vi "Dresden R2R Sputter 03.02.2018 IY24.vi"() -> ()   [LabVIEW 2009] (continued)
                                n31208 = case shown="False" w35965 {
                                tunnel: [FALSE TRUE] -> w35963
                                frame #0 {
                                n31209 = Wait Until Next ms Multiple(millisecond multiple=u32 200) -> ()  [unwired: 1 out]
                                }
                                frame #1 {
                                }
                                }
                                n31210 = Or(x=w35963, y=w35964) -> (x .or. y?=w35962:bool)
                                }
                                }
                                frame #1 {
                                }
                                }
                                }
                                frame #4 {
                                n31211 = local read "Semi"() -> (w35975:bool)
                                n31212 = case shown="False" w35975 {
                                frame #0 {
                                n31213 = local read "Set_pressure_value 2"() -> (w35976:dbl)
                                n31214 = Add(x=1.0, y=w35976) -> (x+y=w35979:dbl)
                                n31215 = Subtract(x=w35976, y=1.0) -> (x-y=w35980:dbl)
                                n31216 = local read "Pressure 2"() -> (w35977:i32)
                                n31217 = In Range and Coerce(upper limit=w35979, x=w35977, lower limit=w35980) -> (In Range?=w35978:bool)  [unwired: 1 out]
                                n31218 = case shown="False" w35978 {
                                frame #0 {
                                n31219 = local read "R Set Pressure mtorr"() -> (w35983:dbl)
                                n31220 = local write "Set_pressure_value 2"(w35983) -> ()
                                }
                                frame #1 {
                                }
                                }
                                }
                                frame #1 {
                                }
                                }
                                }
                                frame #5 {
                                n31221 = local read "Semi"() -> (w35984:bool)
                                n31222 = case shown="False" w35984 {
                                frame #0 {
                                n31223 = local read "Set_pressure_value 2"() -> (w35985:dbl)
                                n31224 = Add(x=1.0, y=w35985) -> (x+y=w35988:dbl)
                                n31225 = Subtract(x=w35985, y=1.0) -> (x-y=w35989:dbl)
                                n31226 = local read "Pressure 2"() -> (w35986:i32)
                                n31227 = In Range and Coerce(upper limit=w35988, x=w35986, lower limit=w35989) -> (In Range?=w35987:bool)  [unwired: 1 out]
                                n31228 = case shown="False" w35987 {
                                frame #0 {
                                n31229 = local write "Pc_bv2_auto_set_pressure"(TRUE ("Pc_bv1_auto_set_pressure")) -> ()
                                }
                                frame #1 {
                                }
                                }
                                }
                                frame #1 {
                                }
                                }
                                }
                                frame #6 {
                                n31230 = local read "Semi"() -> (w35993:bool)
                                n31231 = case shown="False" w35993 {
                                frame #0 {
                                n31232 = while {
                                i -> [w36004]
                                stop <- w35995 stop-if-true
                                n31233 = local read "Set_pressure_value 2"() -> (w35999:dbl)
                                n31234 = Greater?(x=w36004, y=300) -> (0:w35997:bool)
                                n31235 = Add(x=1.0, y=w35999) -> (x+y=w36000:dbl)
                                n31236 = Subtract(x=w35999, y=1.0) -> (x-y=w36001:dbl)
                                n31237 = local read "Pressure 2"() -> (w35994:i32)
                                n31238 = In Range and Coerce(upper limit=w36000, x=w35994, lower limit=w36001) -> (In Range?=w35998:bool)  [unwired: 1 out]
                                n31239 = case shown="False" w35998 {
                                tunnel: [FALSE TRUE] -> w35996
                                frame #0 {
                                n31240 = Wait Until Next ms Multiple(millisecond multiple=u32 200) -> ()  [unwired: 1 out]
                                }
                                frame #1 {
                                }
                                }
                                n31241 = Or(x=w35996, y=w35997) -> (x .or. y?=w35995:bool)
                                }
                                }
                                frame #1 {
                                }
                                }
                                }
                                frame #7 {
                                n31242 = local read "Semi"() -> (w36009:bool)
                                n31243 = case shown="False" w36009 {
                                frame #0 {
                                n31244 = local read "Set_pressure_value 2"() -> (w36012:dbl)
                                n31245 = Add(x=1.0, y=w36012) -> (x+y=w36013:dbl)
                                n31246 = Subtract(x=w36012, y=1.0) -> (x-y=w36014:dbl)
                                n31247 = local read "Pressure 2"() -> (w36010:i32)
                                n31248 = In Range and Coerce(upper limit=w36013, x=w36010, lower limit=w36014) -> (In Range?=w36011:bool)  [unwired: 1 out]
                                n31249 = case shown="False" w36011 {
                                frame #0 {
                                n31250 = local write "Semi"(TRUE ("Semi")) -> ()
                                n31251 = local write "Error Message"("Coating Pressure could not be adjusted !" ("Error Message")) -> ()
                                }
                                frame #1 {
                                }
                                }
                                }
                                frame #1 {
                                }
                                }
                                }
                                }
                                }
                                frame #1 {
                                }
                                }
                                }
                                frame #1 {
                                n31252 = local read "Semi"() -> (w36019:bool)
                                n31253 = case shown="False" w36019 {
                                frame #0 {
                                n31254 = local write "SDC1 9"(TRUE ("SDC1 9")) -> ()
                                n31255 = Wait (ms)(milliseconds to wait=u32 1000) -> ()  [unwired: 1 out]
                                }
                                frame #1 {
                                }
                                }
                                }
                                }
                                }
                                }
                                }
                                frame #1 {
                                }
                                }
                                }
                                frame #13 {
                                n31256 = local read "Semi"() -> (w36022:bool)
                                n31257 = case shown="False" w36022 {
                                frame #0 {
                                n31258 = local write "Start_roll"(TRUE ("Start_roll")) -> ()
                                n31259 = Wait (ms)(milliseconds to wait=u32 300) -> ()  [unwired: 1 out]
                                }
                                frame #1 {
                                }
                                }
                                }
                                frame #14 {
                                n31260 = local read "Semi"() -> (w36025:bool)
                                n31261 = case shown="False" w36025 {
                                frame #0 {
                                n31262 = local read "R Cmb Ch2 Step1 Coating Power Active"() -> (w36036:bool)
                                n31263 = local read "R Cmb Ch2 Step2 Coating Power Active"() -> (w36035:bool)
                                n31264 = local read "R Cmb Ch2 Step3 Coating Power Active"() -> (w36034:bool)
                                n31265 = local read "R Cmb Ch2 Step4 Coating Power Active"() -> (w36033:bool)
                                n31266 = local read "R Cmb Ch2 Step5 Coating Power Active"() -> (w36032:bool)
                                n31267 = Boolean To (0,1)(Boolean=w36036) -> (0, 1=w36031:i16)
                                n31268 = Boolean To (0,1)(Boolean=w36035) -> (0, 1=w36030:i16)
                                n31269 = Boolean To (0,1)(Boolean=w36034) -> (0, 1=w36029:i16)
                                n31270 = Boolean To (0,1)(Boolean=w36033) -> (0, 1=w36028:i16)
                                n31271 = Boolean To (0,1)(Boolean=w36032) -> (0, 1=w36027:i16)
                                n31272 = Compound Arithmetic op=ADD(w36031, w36030, w36029, w36028, w36027) -> (w36026:i16)
                                n31273 = case shown="5" w36026 {
                                frame #0 {
                                }
                                frame #1 {
                                n31274 = stacked-sequence {
                                frame #0 {
                                n31275 = local read "R Cmb Ch2 Step1 Coating Power Active"() -> (w36037:bool)
                                n31276 = case shown="True" w36037 {
                                frame #0 {
                                }
                                frame #1 {
                                n31277 = while {
                                stop <- w36039 stop-if-true
                                n31278 = local read "R Cmb Interval length"() -> (w36043:dbl)
                                n31279 = local read "Actual Length"() -> (w36042:dbl)
                                n31280 = Greater Or Equal?(x=w36042, y=w36043) -> (x >= y?=w36041:bool)
                                n31281 = local read "Semi"() -> (w36040:bool)
                                n31282 = Or(x=w36041, y=w36040) -> (x .or. y?=w36039:bool)
                                n31283 = Wait Until Next ms Multiple(millisecond multiple=u32 300) -> ()  [unwired: 1 out]
                                }
                                }
                                }
                                }
                                }
                                }
                                frame #2 {
                                n31284 = stacked-sequence {
                                frame #0 {
                                n31285 = local read "R Cmb Ch2 Step1 Coating Power Active"() -> (w36044:bool)
                                n31286 = case shown="True" w36044 {
                                frame #0 {
                                }
                                frame #1 {
                                n31287 = while {
                                stop <- w36046 stop-if-true
                                n31288 = local read "R Cmb Interval length"() -> (w36050:dbl)
                                n31289 = local read "Actual Length"() -> (w36049:dbl)
                                n31290 = Greater Or Equal?(x=w36049, y=w36050) -> (x >= y?=w36048:bool)
                                n31291 = local read "Semi"() -> (w36047:bool)
                                n31292 = Or(x=w36048, y=w36047) -> (x .or. y?=w36046:bool)
                                n31293 = Wait Until Next ms Multiple(millisecond multiple=u32 300) -> ()  [unwired: 1 out]
                                }
                                }
                                }
                                }
                                frame #1 {
                                n31294 = local read "R Cmb Ch2 Step2 Coating Power Active"() -> (w36051:bool)
                                n31295 = case shown="True" w36051 {
                                frame #0 {
                                }
                                frame #1 {
                                n31296 = stacked-sequence {
                                frame #0 {
                                n31297 = local read "Semi"() -> (w36052:bool)
                                n31298 = case shown="False" w36052 {
                                frame #0 {
                                n31299 = local read "R Cmb Ch2 Step1 Coating Power"() -> (w36054:dbl)
                                n31300 = Wait (ms)(milliseconds to wait=u32 200) -> ()  [unwired: 1 out]
                                n31301 = local write "Set DC Power       :"(w36054) -> ()
                                }
                                frame #1 {
                                }
                                }
                                }
                                frame #1 {
                                n31302 = local read "Semi"() -> (w36055:bool)
                                n31303 = case shown="False" w36055 {
                                frame #0 {
                                n31304 = local write "Dc_auto_set"(TRUE ("Dc_auto_set")) -> ()
                                }
                                frame #1 {
                                }
                                }
                                }
                                frame #2 {
                                n31305 = while {
                                stop <- w36061 stop-if-true
                                n31306 = local read "R Cmb Interval length"() -> (w36060:dbl)
                                n31307 = local read "Actual Length"() -> (w36064:dbl)
                                n31308 = Multiply(x=w36060, y=2.0) -> (x*y=w36058:dbl)
                                n31309 = Greater Or Equal?(x=w36064, y=w36058) -> (x >= y?=w36063:bool)
                                n31310 = local read "Semi"() -> (w36062:bool)
                                n31311 = Or(x=w36063, y=w36062) -> (x .or. y?=w36061:bool)
                                n31312 = Wait Until Next ms Multiple(millisecond multiple=u32 300) -> ()  [unwired: 1 out]
                                }
                                }
                                }
                                }
                                }
                                }
                                }
                                }
                                frame #3 {
                                n31313 = stacked-sequence {
                                frame #0 {
                                n31314 = local read "R Cmb Ch2 Step1 Coating Power Active"() -> (w36065:bool)
                                n31315 = case shown="True" w36065 {
                                frame #0 {
                                }
                                frame #1 {
                                n31316 = while {
                                stop <- w36067 stop-if-true
                                n31317 = local read "R Cmb Interval length"() -> (w36071:dbl)
                                n31318 = local read "Actual Length"() -> (w36070:dbl)
                                n31319 = Greater Or Equal?(x=w36070, y=w36071) -> (x >= y?=w36069:bool)
                                n31320 = local read "Semi"() -> (w36068:bool)
                                n31321 = Or(x=w36069, y=w36068) -> (x .or. y?=w36067:bool)
                                n31322 = Wait Until Next ms Multiple(millisecond multiple=u32 300) -> ()  [unwired: 1 out]
                                }
                                }
                                }
                                }
                                frame #1 {
                                n31323 = local read "R Cmb Ch2 Step2 Coating Power Active"() -> (w36072:bool)
                                n31324 = case shown="True" w36072 {
                                frame #0 {
                                }
                                frame #1 {
                                n31325 = stacked-sequence {
                                frame #0 {
                                n31326 = local read "Semi"() -> (w36073:bool)
                                n31327 = case shown="False" w36073 {
                                frame #0 {
                                n31328 = local read "R Cmb Ch2 Step2 Coating Power"() -> (w36075:dbl)
                                n31329 = Wait (ms)(milliseconds to wait=u32 200) -> ()  [unwired: 1 out]
                                n31330 = local write "Set DC Power       :"(w36075) -> ()
                                }
                                frame #1 {
                                }
                                }
                                }
                                frame #1 {
                                n31331 = local read "Semi"() -> (w36076:bool)
                                n31332 = case shown="False" w36076 {
                                frame #0 {
                                n31333 = local write "Dc_auto_set"(TRUE ("Dc_auto_set")) -> ()
                                }
                                frame #1 {
                                }
                                }
                                }
                                frame #2 {
                                n31334 = while {
                                stop <- w36082 stop-if-true
                                n31335 = local read "R Cmb Interval length"() -> (w36081:dbl)
                                n31336 = local read "Actual Length"() -> (w36085:dbl)
                                n31337 = Multiply(x=w36081, y=2.0) -> (x*y=w36079:dbl)
                                n31338 = Greater Or Equal?(x=w36085, y=w36079) -> (x >= y?=w36084:bool)
                                n31339 = local read "Semi"() -> (w36083:bool)
                                n31340 = Or(x=w36084, y=w36083) -> (x .or. y?=w36082:bool)
                                n31341 = Wait Until Next ms Multiple(millisecond multiple=u32 300) -> ()  [unwired: 1 out]
                                }
                                }
                                }
                                }
                                }
                                }
                                frame #2 {
                                n31342 = local read "R Cmb Ch2 Step3 Coating Power Active"() -> (w36086:bool)
                                n31343 = case shown="True" w36086 {
                                frame #0 {
                                }
                                frame #1 {
                                n31344 = stacked-sequence {
                                frame #0 {
                                n31345 = local read "Semi"() -> (w36087:bool)
                                n31346 = case shown="False" w36087 {
                                frame #0 {
                                n31347 = local read "R Cmb Ch2 Step1 Coating Power"() -> (w36089:dbl)
                                n31348 = Wait (ms)(milliseconds to wait=u32 200) -> ()  [unwired: 1 out]
                                n31349 = local write "Set DC Power       : 2"(w36089) -> ()
                                }
                                frame #1 {
                                }
                                }
                                }
                                frame #1 {
                                n31350 = local read "Semi"() -> (w36090:bool)
                                n31351 = case shown="False" w36090 {
                                frame #0 {
                                n31352 = local write "Dc_auto_set"(TRUE ("Dc_auto_set")) -> ()
                                }
                                frame #1 {
                                }
                                }
                                }
                                frame #2 {
                                n31353 = while {
                                stop <- w36096 stop-if-true
                                n31354 = local read "R Cmb Interval length"() -> (w36095:dbl)
                                n31355 = local read "Actual Length"() -> (w36099:dbl)
                                n31356 = Multiply(x=w36095, y=3.0) -> (x*y=w36093:dbl)
                                n31357 = Greater Or Equal?(x=w36099, y=w36093) -> (x >= y?=w36098:bool)
                                n31358 = local read "Semi"() -> (w36097:bool)
                                n31359 = Or(x=w36098, y=w36097) -> (x .or. y?=w36096:bool)
                                n31360 = Wait Until Next ms Multiple(millisecond multiple=u32 300) -> ()  [unwired: 1 out]
                                }
                                }
                                }
                                }
                                }
                                }
                                }
                                }
                                frame #4 {
                                n31361 = stacked-sequence {
                                frame #0 {
                                n31362 = local read "R Cmb Ch2 Step1 Coating Power Active"() -> (w36100:bool)
                                n31363 = case shown="True" w36100 {
                                frame #0 {
                                }
                                frame #1 {
                                n31364 = while {
                                stop <- w36102 stop-if-true
                                n31365 = local read "R Cmb Interval length"() -> (w36106:dbl)
                                n31366 = local read "Actual Length"() -> (w36105:dbl)
                                n31367 = Greater Or Equal?(x=w36105, y=w36106) -> (x >= y?=w36104:bool)
                                n31368 = local read "Semi"() -> (w36103:bool)
                                n31369 = Or(x=w36104, y=w36103) -> (x .or. y?=w36102:bool)
                                n31370 = Wait Until Next ms Multiple(millisecond multiple=u32 300) -> ()  [unwired: 1 out]
                                }
                                }
                                }
                                }
                                frame #1 {
                                n31371 = local read "R Cmb Ch2 Step2 Coating Power Active"() -> (w36107:bool)
                                n31372 = case shown="True" w36107 {
                                frame #0 {
                                }
                                frame #1 {
                                n31373 = stacked-sequence {
                                frame #0 {
                                n31374 = local read "Semi"() -> (w36108:bool)
                                n31375 = case shown="False" w36108 {
                                frame #0 {
                                n31376 = local read "R Cmb Ch2 Step3 Coating Power"() -> (w36110:dbl)
                                n31377 = Wait (ms)(milliseconds to wait=u32 200) -> ()  [unwired: 1 out]
                                n31378 = local write "Set DC Power       :"(w36110) -> ()
                                }
                                frame #1 {
                                }
                                }
                                }
                                frame #1 {
                                n31379 = local read "Semi"() -> (w36111:bool)
                                n31380 = case shown="False" w36111 {
                                frame #0 {
                                n31381 = local write "Dc_auto_set"(TRUE ("Dc_auto_set")) -> ()
                                }
                                frame #1 {
                                }
                                }
                                }
                                frame #2 {
                                n31382 = while {
                                stop <- w36117 stop-if-true
                                n31383 = local read "R Cmb Interval length"() -> (w36116:dbl)
                                n31384 = local read "Actual Length"() -> (w36120:dbl)
                                n31385 = Multiply(x=w36116, y=2.0) -> (x*y=w36114:dbl)
                                n31386 = Greater Or Equal?(x=w36120, y=w36114) -> (x >= y?=w36119:bool)
                                n31387 = local read "Semi"() -> (w36118:bool)
                                n31388 = Or(x=w36119, y=w36118) -> (x .or. y?=w36117:bool)
                                n31389 = Wait Until Next ms Multiple(millisecond multiple=u32 300) -> ()  [unwired: 1 out]
                                }
                                }
                                }
                                }
                                }
                                }
                                frame #2 {
                                n31390 = local read "R Cmb Ch2 Step3 Coating Power Active"() -> (w36121:bool)
                                n31391 = case shown="True" w36121 {
                                frame #0 {
                                }
                                frame #1 {
                                n31392 = stacked-sequence {
                                frame #0 {
                                n31393 = local read "Semi"() -> (w36122:bool)
                                n31394 = case shown="False" w36122 {
                                frame #0 {
                                n31395 = local read "R Cmb Ch2 Step2 Coating Power"() -> (w36124:dbl)
                                n31396 = Wait (ms)(milliseconds to wait=u32 200) -> ()  [unwired: 1 out]
                                n31397 = local write "Set DC Power       :"(w36124) -> ()
                                }
                                frame #1 {
                                }
                                }
                                }
                                frame #1 {
                                n31398 = local read "Semi"() -> (w36125:bool)
                                n31399 = case shown="False" w36125 {
                                frame #0 {
                                n31400 = local write "Dc_auto_set"(TRUE ("Dc_auto_set")) -> ()
                                }
                                frame #1 {
                                }
                                }
                                }
                                frame #2 {
                                n31401 = while {
                                stop <- w36131 stop-if-true
                                n31402 = local read "R Cmb Interval length"() -> (w36130:dbl)
                                n31403 = local read "Actual Length"() -> (w36134:dbl)
                                n31404 = Multiply(x=w36130, y=3.0) -> (x*y=w36128:dbl)
                                n31405 = Greater Or Equal?(x=w36134, y=w36128) -> (x >= y?=w36133:bool)
                                n31406 = local read "Semi"() -> (w36132:bool)
                                n31407 = Or(x=w36133, y=w36132) -> (x .or. y?=w36131:bool)
                                n31408 = Wait Until Next ms Multiple(millisecond multiple=u32 300) -> ()  [unwired: 1 out]
                                }
                                }
                                }
                                }
                                }
                                }
                                frame #3 {
                                n31409 = local read "R Cmb Ch2 Step4 Coating Power Active"() -> (w36135:bool)
                                n31410 = case shown="True" w36135 {
                                frame #0 {
                                }
                                frame #1 {
                                n31411 = stacked-sequence {
                                frame #0 {
                                n31412 = local read "Semi"() -> (w36136:bool)
                                n31413 = case shown="False" w36136 {
                                frame #0 {
                                n31414 = local read "R Cmb Ch2 Step1 Coating Power"() -> (w36138:dbl)
                                n31415 = Wait (ms)(milliseconds to wait=u32 200) -> ()  [unwired: 1 out]
                                n31416 = local write "Set DC Power       :"(w36138) -> ()
                                }
                                frame #1 {
                                }
                                }
                                }
                                frame #1 {
                                n31417 = local read "Semi"() -> (w36139:bool)
                                n31418 = case shown="False" w36139 {
                                frame #0 {
                                n31419 = local write "Dc_auto_set"(TRUE ("Dc_auto_set")) -> ()
                                }
                                frame #1 {
                                }
                                }
                                }
                                frame #2 {
                                n31420 = while {
                                stop <- w36145 stop-if-true
                                n31421 = local read "R Cmb Interval length"() -> (w36144:dbl)
                                n31422 = local read "Actual Length"() -> (w36148:dbl)
                                n31423 = Multiply(x=w36144, y=4.0) -> (x*y=w36142:dbl)
                                n31424 = Greater Or Equal?(x=w36148, y=w36142) -> (x >= y?=w36147:bool)
                                n31425 = local read "Semi"() -> (w36146:bool)
                                n31426 = Or(x=w36147, y=w36146) -> (x .or. y?=w36145:bool)
                                n31427 = Wait Until Next ms Multiple(millisecond multiple=u32 300) -> ()  [unwired: 1 out]
                                }
                                }
                                }
                                }
                                }
                                }
                                }
                                }
                                frame #5 {
                                n31428 = stacked-sequence {
                                frame #0 {
                                n31429 = local read "R Cmb Ch2 Step1 Coating Power Active"() -> (w36149:bool)
                                n31430 = case shown="True" w36149 {
                                frame #0 {
                                }
                                frame #1 {
                                n31431 = while {
                                stop <- w36151 stop-if-true
                                n31432 = local read "R Cmb Interval length"() -> (w36155:dbl)
                                n31433 = local read "Actual Length"() -> (w36154:dbl)
                                n31434 = Greater Or Equal?(x=w36154, y=w36155) -> (x >= y?=w36153:bool)
                                n31435 = local read "Semi"() -> (w36152:bool)
                                n31436 = Or(x=w36153, y=w36152) -> (x .or. y?=w36151:bool)
                                n31437 = Wait Until Next ms Multiple(millisecond multiple=u32 300) -> ()  [unwired: 1 out]
                                }
                                }
                                }
                                }
                                frame #1 {
                                n31438 = local read "R Cmb Ch2 Step2 Coating Power Active"() -> (w36156:bool)
                                n31439 = case shown="True" w36156 {
                                frame #0 {
                                }
                                frame #1 {
                                n31440 = stacked-sequence {
                                frame #0 {
                                n31441 = local read "Semi"() -> (w36157:bool)
                                n31442 = case shown="False" w36157 {
                                frame #0 {
                                n31443 = local read "R Cmb Ch2 Step4 Coating Power"() -> (w36159:dbl)
                                n31444 = Wait (ms)(milliseconds to wait=u32 200) -> ()  [unwired: 1 out]
                                n31445 = local write "Set DC Power       :"(w36159) -> ()
                                }
                                frame #1 {
                                }
                                }
                                }
                                frame #1 {
                                n31446 = local read "Semi"() -> (w36160:bool)
                                n31447 = case shown="False" w36160 {
                                frame #0 {
                                n31448 = local write "Dc_auto_set"(TRUE ("Dc_auto_set")) -> ()
                                }
                                frame #1 {
                                }
                                }
                                }
                                frame #2 {
                                n31449 = while {
                                stop <- w36166 stop-if-true
                                n31450 = local read "R Cmb Interval length"() -> (w36165:dbl)
                                n31451 = local read "Actual Length"() -> (w36169:dbl)
                                n31452 = Multiply(x=w36165, y=2.0) -> (x*y=w36163:dbl)
                                n31453 = Greater Or Equal?(x=w36169, y=w36163) -> (x >= y?=w36168:bool)
                                n31454 = local read "Semi"() -> (w36167:bool)
                                n31455 = Or(x=w36168, y=w36167) -> (x .or. y?=w36166:bool)
                                n31456 = Wait Until Next ms Multiple(millisecond multiple=u32 300) -> ()  [unwired: 1 out]
                                }
                                }
                                }
                                }
                                }
                                }
                                frame #2 {
                                n31457 = local read "R Cmb Ch2 Step3 Coating Power Active"() -> (w36170:bool)
                                n31458 = case shown="True" w36170 {
                                frame #0 {
                                }
                                frame #1 {
                                n31459 = stacked-sequence {
                                frame #0 {
                                n31460 = local read "Semi"() -> (w36171:bool)
                                n31461 = case shown="False" w36171 {
                                frame #0 {
                                n31462 = local read "R Cmb Ch2 Step3 Coating Power"() -> (w36173:dbl)
                                n31463 = Wait (ms)(milliseconds to wait=u32 200) -> ()  [unwired: 1 out]
                                n31464 = local write "Set DC Power       :"(w36173) -> ()
                                }
                                frame #1 {
                                }
                                }
                                }
                                frame #1 {
                                n31465 = local read "Semi"() -> (w36174:bool)
                                n31466 = case shown="False" w36174 {
                                frame #0 {
                                n31467 = local write "Dc_auto_set"(TRUE ("Dc_auto_set")) -> ()
                                }
                                frame #1 {
                                }
                                }
                                }
                                frame #2 {
                                n31468 = while {
                                stop <- w36180 stop-if-true
                                n31469 = local read "R Cmb Interval length"() -> (w36179:dbl)
                                n31470 = local read "Actual Length"() -> (w36183:dbl)
                                n31471 = Multiply(x=w36179, y=3.0) -> (x*y=w36177:dbl)
                                n31472 = Greater Or Equal?(x=w36183, y=w36177) -> (x >= y?=w36182:bool)
                                n31473 = local read "Semi"() -> (w36181:bool)
                                n31474 = Or(x=w36182, y=w36181) -> (x .or. y?=w36180:bool)
                                n31475 = Wait Until Next ms Multiple(millisecond multiple=u32 300) -> ()  [unwired: 1 out]
                                }
                                }
                                }
                                }
                                }
                                }
                                frame #3 {
                                n31476 = local read "R Cmb Ch2 Step4 Coating Power Active"() -> (w36184:bool)
                                n31477 = case shown="True" w36184 {
                                frame #0 {
                                }
                                frame #1 {
                                n31478 = stacked-sequence {
                                frame #0 {
                                n31479 = local read "Semi"() -> (w36185:bool)
                                n31480 = case shown="False" w36185 {
                                frame #0 {
                                n31481 = local read "R Cmb Ch2 Step2 Coating Power"() -> (w36187:dbl)
                                n31482 = Wait (ms)(milliseconds to wait=u32 200) -> ()  [unwired: 1 out]
                                n31483 = local write "Set DC Power       :"(w36187) -> ()
                                }
                                frame #1 {
                                }
                                }
                                }
                                frame #1 {
                                n31484 = local read "Semi"() -> (w36188:bool)
                                n31485 = case shown="False" w36188 {
                                frame #0 {
                                n31486 = local write "Dc_auto_set"(TRUE ("Dc_auto_set")) -> ()
                                }
                                frame #1 {
                                }
                                }
                                }
                                frame #2 {
                                n31487 = while {
                                stop <- w36194 stop-if-true
                                n31488 = local read "R Cmb Interval length"() -> (w36193:dbl)
                                n31489 = local read "Actual Length"() -> (w36197:dbl)
                                n31490 = Multiply(x=w36193, y=4.0) -> (x*y=w36191:dbl)
                                n31491 = Greater Or Equal?(x=w36197, y=w36191) -> (x >= y?=w36196:bool)
                                n31492 = local read "Semi"() -> (w36195:bool)
                                n31493 = Or(x=w36196, y=w36195) -> (x .or. y?=w36194:bool)
                                n31494 = Wait Until Next ms Multiple(millisecond multiple=u32 300) -> ()  [unwired: 1 out]
                                }
                                }
                                }
                                }
                                }
                                }
                                frame #4 {
                                n31495 = local read "R Cmb Ch2 Step5 Coating Power Active"() -> (w36198:bool)
                                n31496 = case shown="True" w36198 {
                                frame #0 {
                                }
                                frame #1 {
                                n31497 = stacked-sequence {
                                frame #0 {
                                n31498 = local read "Semi"() -> (w36199:bool)
                                n31499 = case shown="False" w36199 {
                                frame #0 {
                                n31500 = local read "R Cmb Ch2 Step1 Coating Power"() -> (w36201:dbl)
                                n31501 = Wait (ms)(milliseconds to wait=u32 200) -> ()  [unwired: 1 out]
                                n31502 = local write "Set DC Power       :"(w36201) -> ()
                                }
                                frame #1 {
                                }
                                }
                                }
                                frame #1 {
                                n31503 = local read "Semi"() -> (w36202:bool)
                                n31504 = case shown="False" w36202 {
                                frame #0 {
                                n31505 = local write "Dc_auto_set"(TRUE ("Dc_auto_set")) -> ()
                                }
                                frame #1 {
                                }
                                }
                                }
                                frame #2 {
                                n31506 = while {
                                stop <- w36208 stop-if-true
                                n31507 = local read "R Cmb Interval length"() -> (w36207:dbl)
                                n31508 = local read "Actual Length"() -> (w36211:dbl)
                                n31509 = Multiply(x=w36207, y=5.0) -> (x*y=w36205:dbl)
                                n31510 = Greater Or Equal?(x=w36211, y=w36205) -> (x >= y?=w36210:bool)
                                n31511 = local read "Semi"() -> (w36209:bool)
                                n31512 = Or(x=w36210, y=w36209) -> (x .or. y?=w36208:bool)
                                n31513 = Wait Until Next ms Multiple(millisecond multiple=u32 300) -> ()  [unwired: 1 out]
                                }
                                }
                                }
                                }
                                }
                                }
                                }
                                }
                                }
                                }
                                frame #1 {
                                }
                                }
                                }
                                frame #15 {
                                n31514 = local read "Semi"() -> (w36212:bool)
                                n31515 = case shown="False" w36212 {
                                frame #0 {
                                n31516 = local write "SDC1 13b"(TRUE ("SDC1 13b")) -> ()
                                n31517 = Wait (ms)(milliseconds to wait=u32 1000) -> ()  [unwired: 1 out]
                                }
                                frame #1 {
                                }
                                }
                                }
                                }
                                }
                                frame #1 {
                                }
                                }
                                }
                                frame #13 {
                                # "CLOSE DC"
                                n31518 = local read "Semi"() -> (w36215:bool)
                                n31519 = case shown="False" w36215 {
                                frame #0 {
                                n31520 = stacked-sequence {
                                frame #0 {
                                n31521 = local read "Semi"() -> (w36216:bool)
                                n31522 = case shown="False" w36216 {
                                frame #0 {
                                n31523 = local write "Dc_auto_off"(TRUE ("Dc_auto_off")) -> ()
                                }
                                frame #1 {
                                }
                                }
                                }
                                frame #1 {
                                n31524 = local read "Semi"() -> (w36218:bool)
                                n31525 = case shown="False" w36218 {
                                frame #0 {
                                n31526 = Wait (ms)(milliseconds to wait=u32 1000) -> ()  [unwired: 1 out]